vi "HFRR ADV v039.vi"() -> ()   [LabVIEW 2025] (continued)
            n1308 = Not(x=w1623) -> (.not. x?=w1622:bool)
            n1309 = local write "CAMERA ROI MIN TEMP"(w1622) -> ()
            n1310 = call "IMAGE ANALYSIS.vi"("Enum"=POST_ANALYSIS_ENUM."MINIMIZE UI") -> ()  [unwired: 9 in, 2 out]
          }
        }
        n1311 = local write "CAMERA ROI MAX TEMP"(TRUE ("CAMERA ROI MIN TEMP")) -> ()
      }
      frame "Advance" {
        n1312 = local read "LIVE FEED MIN TEMP"() -> (w1629:bool)
        n1313 = local write "LIVE FEED MAX TEMP"(TRUE ("LIVE FEED MAX TEMP")) -> ()
        n1314 = local read "CAMERA ROI MIN TEMP"() -> (w1627:bool)
        n1315 = case shown="True" w1629 {
          selector: w1629 -> [_ w1636]
          frame False {
          }
          frame True {
            n1316 = Not(x=w1636) -> (.not. x?=w1635:bool)
            n1317 = local write "LIVE FEED MIN TEMP"(w1635) -> ()
            n1318 = call "CAMERA LIVE FEED FGV.vi"("Enum - Menu"=CAMERA_LIVE_FEED_ENUM."CAMERA MINIMIZE") -> ()  [unwired: 9 in, 2 out]
          }
        }
        n1319 = local write "CAMERA ROI MAX TEMP"(TRUE ("CAMERA ROI MAX TEMP")) -> ()
        n1320 = case shown="True" w1627 {
          selector: w1627 -> [_ w1633]
          frame False {
          }
          frame True {
            n1321 = Not(x=w1633) -> (.not. x?=w1632:bool)
            n1322 = local write "CAMERA ROI MIN TEMP"(w1632) -> ()
            n1323 = call "IMAGE ANALYSIS.vi"("Enum"=POST_ANALYSIS_ENUM."MINIMIZE UI") -> ()  [unwired: 9 in, 2 out]
          }
        }
      }
      frame "Mooha" {
        n1324 = local read "LIVE FEED MIN TEMP"() -> (w1639:bool)
        n1325 = local write "LIVE FEED MAX TEMP"(TRUE ("LIVE FEED MAX TEMP")) -> ()
        n1326 = local read "CAMERA ROI MIN TEMP"() -> (w1637:bool)
        n1327 = case shown="True" w1639 {
          selector: w1639 -> [_ w1646]
          frame False {
          }
          frame True {
            n1328 = Not(x=w1646) -> (.not. x?=w1645:bool)
            n1329 = local write "LIVE FEED MIN TEMP"(w1645) -> ()
            n1330 = call "CAMERA LIVE FEED FGV.vi"("Enum - Menu"=CAMERA_LIVE_FEED_ENUM."CAMERA MINIMIZE") -> ()  [unwired: 9 in, 2 out]
          }
        }
        n1331 = local write "CAMERA ROI MAX TEMP"(TRUE ("CAMERA ROI MAX TEMP")) -> ()
        n1332 = case shown="True" w1637 {
          selector: w1637 -> [_ w1643]
          frame False {
          }
          frame True {
            n1333 = Not(x=w1643) -> (.not. x?=w1642:bool)
            n1334 = local write "CAMERA ROI MIN TEMP"(w1642) -> ()
            n1335 = call "IMAGE ANALYSIS.vi"("Enum"=POST_ANALYSIS_ENUM."MINIMIZE UI") -> ()  [unwired: 9 in, 2 out]
          }
        }
      }
    }
    n1336 = local read "Auto Start Test"() -> (w1384:bool)
    n1337 = case shown="True" "sign in temp" {
      frame False {
      }
      frame True {
        w1419 = 1 ("y")
        n1338 = local read "USERNAME"() -> (w1425:string)
        n1339 = local read "USER ID"() -> (w1422:string)
        n1340 = call <vilib>:"Trim Whitespace.vi"("string"=w1425) -> ("trimmed string"=w1424:string)  [unwired: 1 in]
        n1341 = call <vilib>:"Trim Whitespace.vi"("string"=w1422) -> ("trimmed string"=w1423:string)  [unwired: 1 in]
        n1342 = String Length(string=w1424) -> (length=w1421:i32)
        n1343 = String Length(string=w1423) -> (length=w1420:i32)
        n1344 = Greater?(x=w1421, y=w1419) -> (0:w1418:bool)
        n1345 = Greater?(x=w1420, y=w1419) -> (0:w1417:bool)
        n1346 = And(x=w1418, y=w1417) -> (x .and. y?=w1416:bool)
        n1347 = case shown="True" w1416 {
          frame False {
            n1348 = property on="Sign In" class="Bool (strict)"("DisabledEnum"=T19."Disabled" ("Disabled")) -> ()  [unwired: 2 in, 2 out]
          }
          frame True {
            n1349 = property on="Sign In" class="Bool (strict)"("DisabledEnum"=T19."Enabled" ("Disabled")) -> ()  [unwired: 2 in, 2 out]
          }
        }
      }
    }
    n1350 = local read "Air Temperature"() -> (w1401:bool)
    n1351 = local read "Coefficient Of Friction"() -> (w1402:bool)
    n1352 = case shown="False" w1384 {
      frame False {
        n1353 = local read "Auto stop temp"() -> (w1413:bool)
        n1354 = case shown="True" w1413 {
          frame False {
          }
          frame True {
            n1355 = local write "Auto Start Temp"(FALSE ("Auto Start Temp")) -> ()
          }
        }
      }
      frame True {
        "Auto stop temp" <- TRUE ("Auto stop temp")
      }
    }
    n1356 = local read "Humidity"() -> (w1400:bool)
    n1357 = case shown="\"HOME\"" w1410 {
      frame "HOME" {
        n1358 = local write "main tab sub"(enum32{"Page 1", "Page 2"}."Page 1" ("main tab sub")) -> ()
      }
      frame Default {
        n1359 = local write "main tab sub"(enum32{"Page 1", "Page 2"}."Page 2" ("main tab sub")) -> ()
      }
    }
    n1360 = case shown="True" w1409 {
      selector: w1409 -> [_ w1761]
      frame False {
      }
      frame True {
        n1361 = Not(x=w1761) -> (.not. x?=w1760:bool)
        n1362 = local write "Sign In"(w1760) -> ()
        n1363 = local write "Main Dashboard Buttons"(T26."Test Setup" ("Main Dashboard Buttons")) -> ()
      }
    }
    n1364 = case shown="\"Numeric Display\", Default" "Num/Graph" {
      frame "Numeric Display", Default {
        n1365 = property on="Single/Multiple" class="RadioBtnsControl (strict)"("Visible"=FALSE) -> ()  [unwired: 2 in, 2 out]
        n1366 = property on="Single - Graph" class="Ring (strict)"("Visible"=FALSE) -> ()  [unwired: 2 in, 2 out]
        n1367 = local write "Main Tab Display"(T4."Dashboard 1" ("Main Tab Display")) -> ()
      }
      frame "Graph Display" {
        n1368 = property on="Single/Multiple" class="RadioBtnsControl (strict)"("Visible"=TRUE) -> ()  [unwired: 2 in, 2 out]
        n1369 = case shown="\"Multiple\"" "Single/Multiple" {
          frame "Single ", Default {
            n1370 = property on="Single - Graph" class="Ring (strict)"("Visible"=TRUE) -> ()  [unwired: 2 in, 2 out]
            n1371 = local write "Main Tab Display"(T4."Dashboard 3" ("Main Tab Display")) -> ()
          }
          frame "Multiple" {
            n1372 = property on="Single - Graph" class="Ring (strict)"("Visible"=FALSE) -> ()  [unwired: 2 in, 2 out]
            n1373 = local write "Main Tab Display"(T4."Dashboard 2" ("Main Tab Display")) -> ()
          }
        }
      }
    }
    n1374 = local read "Stroke"() -> (w1399:bool)
    n1375 = local read "USERNAME"() -> (w1404:string)
    n1376 = case shown="True" w1402 {
      selector: w1402 -> [_ w1686]
      frame False {
      }
      frame True {
        n1377 = Not(x=w1686) -> (.not. x?=w1685:bool)
        n1378 = local write "Coefficient Of Friction"(w1685) -> ()
        n1379 = local write "Tab Control 2"(T6."Coefficient Of Friction" ("Tab Control 2")) -> ()
      }
    }
    n1380 = case shown="True" w1401 {
      selector: w1401 -> [_ w1683]
      frame False {
      }
      frame True {
        n1381 = Not(x=w1683) -> (.not. x?=w1681:bool)
        n1382 = local write "Air Temperature"(w1681) -> ()
        n1383 = local write "Tab Control 2"(T6."Air Temperature" ("Tab Control 2")) -> ()
      }
    }
    n1384 = case shown="True" w1399 {
      selector: w1399 -> [_ w1677]
      frame False {
      }
      frame True {
        n1385 = Not(x=w1677) -> (.not. x?=w1675:bool)
        n1386 = local write "Stroke"(w1675) -> ()
        n1387 = local write "Tab Control 2"(T6."Stroke" ("Tab Control 2")) -> ()
      }
    }
    n1388 = local write "tested by"(w1404) -> ()
    n1389 = case shown="True" w1400 {
      selector: w1400 -> [_ w1680]
      frame False {
      }
      frame True {
        n1390 = Not(x=w1680) -> (.not. x?=w1678:bool)
        n1391 = local write "Humidity"(w1678) -> ()
        n1392 = local write "Tab Control 2"(T6."Humidity" ("Tab Control 2")) -> ()
      }
    }
    n1393 = case shown="\"Calibration\"" "Main Dashboard Buttons" {
      tunnel: [T2."HOME" ("Main Tab") T2."Test Setup" ("Main Tab") T2."Acquire" ("Main Tab") T2."Adv Scar" ("Main Tab") T2."Adv Scar Report" ("Main Tab") T2."Compare Files" ("Main Tab") T2."Calibration" ("Main Tab") T2."About" ("Main Tab") T2."Advance" ("Main Tab")] -> w1383
      frame "Home", Default {
      }
      frame "Test Setup" {
      }
      frame "Dashboard" {
      }
      frame "Imaging" {
      }
      frame "Report" {
      }
      frame "Analysis" {
      }
      frame "Calibration" {
      }
      frame "About" {
      }
      frame "Advance" {
      }
    }
    n1394 = Wait (ms)(milliseconds to wait=u32 100) -> ()  [unwired: 1 out]
    n1395 = local read "Main Tab Display"() -> (w1403:T4)
    n1396 = local write "Main Tab"(w1383) -> ()
    n1397 = case shown="\"Dashboard 3\"" w1403 {
      frame "Dashboard 1", Default {
        n1398 = property on="Reset Graph" class="Bool (strict)"("Visible"=FALSE) -> ()  [unwired: 2 in, 2 out]
      }
      frame "Dashboard 2" {
        n1399 = property on="Reset Graph" class="Bool (strict)"("Visible"=TRUE) -> ()  [unwired: 2 in, 2 out]
      }
      frame "Dashboard 3" {
        n1400 = property on="Reset Graph" class="Bool (strict)"("Visible"=TRUE) -> ()  [unwired: 2 in, 2 out]
      }
    }
    n1401 = local read "SCAR MEASURMENT"() -> (w1391:enum32{"Auto Scar", "Manual Scar"})
    n1402 = local read "Humidity"() -> (w1405:bool)
    n1403 = local read "Cap Live Image"() -> (w1388:bool)
    n1404 = local read "Sample Temperature"() -> (w1398:bool)
    n1405 = local read "Air Temp vs Humidity"() -> (w1396:bool)
    n1406 = local read "Frequency"() -> (w1397:bool)
    n1407 = case shown="False" w1405 {
      frame False {
        n1408 = local write "Humidity On Command"(TRUE ("Humidity On Command")) -> ()
        n1409 = case shown="True" "Humidity Off Command" {
          selector: "Humidity Off Command" -> [_ w1693]
          frame False {
          }
          frame True {
            n1410 = stacked-sequence {
              frame #0 {
                n1411 = local read "WriteHumidity"() -> (w1695:string[])
                n1412 = Insert Into Array(array=w1695, new element="R;1" ("new element/subarray")) -> (w1694:string[])  [unwired: 1 in]
                n1413 = local write "WriteHumidity"(w1694) -> ()
              }
              frame #1 {
                n1414 = Wait (ms)(milliseconds to wait=u32 500) -> ()  [unwired: 1 out]
              }
              frame #2 {
                n1415 = local read "WriteHumidity"() -> (w1699:string[])
                n1416 = local read "EVENT LOG"() -> (w1703:string)
                n1417 = call "Event Log.vi"("Content"="Humidity Control Off" ("string"), "EVENT LOG"=w1703) -> ("EVENT LOG"=w1704:string)  [unwired: 8 in, 1 out]
                n1418 = local write "EVENT LOG"(w1704) -> ()
                n1419 = Insert Into Array(array=w1699, new element="R;1" ("new element/subarray")) -> (w1700:string[])  [unwired: 1 in]
                n1420 = local write "WriteHumidity"(w1700) -> ()
                n1421 = local write "Humidity 2"(TRUE ("Humidity")) -> ()
              }
            }
            n1422 = Not(x=w1693) -> (.not. x?=w1692:bool)
            n1423 = local write "Humidity Off Command"(w1692) -> ()
          }
        }
      }
      frame True {
        n1424 = local write "Humidity Off Command"(TRUE ("Humidity Off Command")) -> ()
        n1425 = case shown="False" "Humidity On Command" {
          selector: "Humidity On Command" -> [_ w1708]
          frame False {
          }
          frame True {
            n1426 = stacked-sequence {
              frame #0 {
                n1427 = local read "Set Rh"() -> (w1714:dbl)
                n1428 = local read "WriteHumidity"() -> (w1710:string[])
                n1429 = Number To Fractional String(number=w1714, precision (6)=i16 2) -> (F-format string=w1715:string)  [unwired: 2 in]
                n1430 = Concatenate Strings("M;" ("new element/subarray"), w1715) -> (w1713:string)
                n1431 = Insert Into Array(array=w1710, new element=w1713) -> (w1709:string[])  [unwired: 1 in]
                n1432 = local write "WriteHumidity"(w1709) -> ()
              }
              frame #1 {
                n1433 = Wait (ms)(milliseconds to wait=u32 500) -> ()  [unwired: 1 out]
              }
              frame #2 {
                n1434 = local read "WriteHumidity"() -> (w1718:string[])
                n1435 = local read "Set Rh"() -> (w1722:dbl)
                n1436 = Number To Fractional String(number=w1722, precision (6)=i16 2) -> (F-format string=w1723:string)  [unwired: 2 in]
                n1437 = Concatenate Strings("M;" ("new element/subarray"), w1723) -> (w1721:string)
                n1438 = Insert Into Array(array=w1718, new element=w1721) -> (w1717:string[])  [unwired: 1 in]
                n1439 = local write "WriteHumidity"(w1717) -> ()
              }
              frame #3 {
                n1440 = Wait (ms)(milliseconds to wait=u32 500) -> ()  [unwired: 1 out]
              }
              frame #4 {
                (unwired) "% RH" ("string")
                (unwired) i16 2 ("precision (6)")
                (unwired) "M;" ("new element/subarray")
                n1441 = local read "Set Rh"() -> (w1732:dbl)
                n1442 = local read "WriteHumidity"() -> (w1725:string[])
                n1443 = Number To Fractional String(number=w1732, precision (6)=i16 2) -> (F-format string=w1729:string)  [unwired: 2 in]
                n1444 = Concatenate Strings("M;" ("new element/subarray"), w1729) -> (w1733:string)
                n1445 = Concatenate Strings("Humidity Set to : " ("string"), w1729, "% RH" ("string")) -> (w1727:string)
                n1446 = Insert Into Array(array=w1725, new element=w1733) -> (w1726:string[])  [unwired: 1 in]
                n1447 = disable-structure shown="Enabled" {
                  frame Enabled {
                    n1448 = local read "EVENT LOG"() -> (w1736:string)
                    n1449 = call "Event Log.vi"("Content"="Humidity Control On", "EVENT LOG"=w1736) -> ("EVENT LOG"=w1737:string)  [unwired: 8 in, 1 out]
                    n1450 = local write "EVENT LOG"(w1737) -> ()
                  }
                  frame Disabled {
                  }
                }
                n1451 = disable-structure shown="Enabled" {
                  disable-tunnel: w1727 -> [_ _]
                  frame Enabled {
                    n1452 = local read "EVENT LOG"() -> (w1739:string)
                    n1453 = call "Event Log.vi"("Content"="Humidity Control On", "EVENT LOG"=w1739) -> ("EVENT LOG"=w1740:string)  [unwired: 8 in, 1 out]
                    n1454 = local write "EVENT LOG"(w1740) -> ()
                  }
                  frame Disabled {
                  }
                }
                n1455 = local write "WriteHumidity"(w1726) -> ()
              }
            }
            n1456 = Not(x=w1708) -> (.not. x?=w1707:bool)
            n1457 = local write "Humidity On Command"(w1707) -> ()
          }
        }
      }
    }
    n1458 = Equal?(x=w1391, y=enum32{"Auto Scar", "Manual Scar"}."Auto Scar" ("SCAR MEASURMENT")) -> (x = y?=w1387:bool)
    n1459 = local read "TEST STANDARD"() -> (w1394:T3)
    n1460 = And(x=w1388, y=w1387) -> (x .and. y?=w1389:bool)
    n1461 = case shown="True" w1389 {
      selector: w1389 -> [_ w1492]
      tunnel: errorcluster {"status"=FALSE, "code"=0, "source"=""} ("error in (no error) 3") -> [_ w1493]
      frame False {
      }
      frame True {
        n1462 = stacked-sequence {
          tunnel: w1493 -> [_ _ _ _ _ _ _ w1541]
          tunnel: w1492 -> [_ _ _ _ _ w1522 _ _]
          frame #0 {
            n1463 = call "CAMERA LIVE FEED FGV.vi"("Enum - Menu"=CAMERA_LIVE_FEED_ENUM."CAMERA MINIMIZE") -> ()  [unwired: 9 in, 2 out]
          }
          frame #1 {
            n1464 = property on="Auto Scar Check  2" class="Clust (strict)"("Visible"=TRUE) -> ()  [unwired: 2 in, 2 out]
          }
          frame #2 {
            n1465 = String To Path(string="C:\\LAB-IQ\\Image Calibrate v01.dcf") -> (path=w1498:path)
            n1466 = Open/Create/Replace File ("Open File")(file path (use dialog)=w1498) -> (refnum out=w1499:refnum<file>)  [unwired: 5 in, 2 out]
            n1467 = for {
              N: 4 -> [_]
              tunnel: w1499 -> [w1505]
              i -> [w1501]
              n1468 = Read from Text File ("Read File")(file (use dialog)=w1505) -> (text=w1506:string)  [unwired: 3 in, 3 out]
              n1469 = String Subset(string=w1506, offset (0)=6, length (rest)=10 ("length (rest)")) -> (substring=w1502:string)
              n1470 = Fract/Exp String To Number(string=w1502) -> (number=w1500:dbl)  [unwired: 3 in, 1 out]
              n1471 = case shown="0" w1501 {
                tunnel: w1500 -> [w1507 w1508 _ w1509 _]
                frame 0 {
                  "5x Gain" <- w1507
                }
                frame 1 {
                  "10x Gain" <- w1508
                }
                frame 2 {
                }
                frame 3 {
                  "100x gain" <- w1509
                }
                frame 4, Default {
                }
              }
            }
          }
          frame #3 {
            n1472 = local read "FILE 3"() -> (w1515:string)
            n1473 = call <vilib>:"Trim Whitespace.vi"("string"="C:\\LAB-IQ\\images\\") -> ("trimmed string"=w1517:string)  [unwired: 1 in]
            n1474 = String To Path(string=w1517) -> (path=w1516:path)
            n1475 = Concatenate Strings(w1515, ".png" ("string")) -> (w1514:string)
            n1476 = Build Path(base path=w1516, name or relative path=w1514) -> (appended path=w1512:path)
            "Image path" <- w1512
            n1477 = Path To String(path=w1512) -> (string=w1511:string)
            n1478 = call "CAMERA LIVE FEED FGV.vi"("Enum - Menu"=CAMERA_LIVE_FEED_ENUM."CAMERA SAVE", "Image Path"=w1511) -> ()  [unwired: 8 in, 2 out]
          }
          frame #4 {
            n1479 = One Button Dialog(message="Image saved successfully") -> ()  [unwired: 1 in, 1 out]
          }
          frame #5 {
            n1480 = local read "TEST STANDARD"() -> (w1521:T3)
            n1481 = local read "Magnification len live scar"() -> (w1533:string)
            n1482 = Not(x=w1522) -> (.not. x?=w1523:bool)
            n1483 = local write "Cap Live Image"(w1523) -> ()
            n1484 = case shown="\"ISO 12156\"" w1521 {
              tunnel: ["ASTM D6079" "ISO 12156"] -> w1520
              frame "ASTM D6079", Default {
              }
              frame "ISO 12156" {
              }
            }
            n1485 = case shown="\"5x\", Default" w1533 {
              tunnel: [w1536 w1537] -> w1532
              frame "5x", Default {
                n1486 = local read "5x Gain"() -> (w1536:dbl)
              }
              frame "10x" {
                # "5x"
                n1487 = local read "10x Gain"() -> (w1537:dbl)
              }
            }
            n1488 = local read "Image path"() -> (w1531:path)
            n1489 = local read "FILE 3"() -> (w1524:string)
            n1490 = call "EDGE DETCTION.vi"("GAIN VALUE"=w1532, "Image Path"=w1531) -> ("error out"=w1530:errorcluster, "return value"=w1529:cluster{string, string, dbl, dbl, dbl})  [unwired: 8 in]
            n1491 = Bundle By Name(cluster=T27 {"File Name"="", "Test Method"="", "Operator"="", "Fuel Description"="", "Date and time"=""} ("Main Ref"), "File Name"=w1524, "Test Method"=w1520) -> (w1525:T27)
            n1492 = call "duf file read.vi"("error in (no error)"=w1530, "Main Ref"=w1525) -> ("error out"=w1528:errorcluster, "Main Ref 2"=w1526:T27)  [unwired: 8 in]
            n1493 = call "EDGE DETECTION REPORT.vi"("error in (no error)"=w1528, "return value 2"=w1529, "Main Ref"=w1526) -> ()  [unwired: 8 in, 1 out]
          }
          frame #6 {
            n1494 = property on="Auto Scar Check  2" class="Clust (strict)"("Visible"=FALSE) -> ()  [unwired: 2 in, 2 out]
          }
          frame #7 {
            n1495 = call "CAMERA LIVE FEED FGV.vi"("Enum - Menu"=CAMERA_LIVE_FEED_ENUM."CAMERA MINIMIZE", "error in (no error)"=w1541) -> ()  [unwired: 8 in, 2 out]
            n1496 = local write "Main Dashboard Buttons"(T1."Home" ("Main Dashboard Buttons")) -> ()
            n1497 = local write "Main Tab"(T2."HOME" ("Main Tab")) -> ()
          }
        }
      }
    }
    n1498 = local read "Heater Button"() -> (w1395:bool)
    n1499 = case shown="True" w1397 {
      selector: w1397 -> [_ w1671]
      frame False {
      }
      frame True {
        n1500 = Not(x=w1671) -> (.not. x?=w1669:bool)
        n1501 = local write "Frequency"(w1669) -> ()
        n1502 = local write "Tab Control 2"(T6."Frequency" ("Tab Control 2")) -> ()
      }
    }
    n1503 = case shown="True" w1396 {
      selector: w1396 -> [_ w1668]
      frame False {
      }
      frame True {
        n1504 = Not(x=w1668) -> (.not. x?=w1666:bool)
        n1505 = local write "Air Temp vs Humidity"(w1666) -> ()
        n1506 = local write "Tab Control 2"(T6."Air Temp vs Rh" ("Tab Control 2")) -> ()
      }
    }
    n1507 = case shown="True" w1398 {
      selector: w1398 -> [_ w1674]
      frame False {
      }
      frame True {
        n1508 = Not(x=w1674) -> (.not. x?=w1672:bool)
        n1509 = local write "Sample Temperature"(w1672) -> ()
        n1510 = local write "Tab Control 2"(T6."Sample Temperature" ("Tab Control 2")) -> ()
      }
    }
    n1511 = case shown="\"Custom\"" w1394 {
      frame "ASTM D6079", Default {
        w1647 = "ASTM D6079 TEST CONDITIONS" ("Standard 2")
        n1512 = local write "Standard 2"(w1647) -> ()
        n1513 = local write "Standard"(w1647) -> ()
      }
      frame "ISO 12156" {
        w1648 = "ISO 12156 TEST CONDITIONS" ("Standard 2")
        n1514 = local write "Standard 2"(w1648) -> ()
        n1515 = local write "Standard"(w1648) -> ()
      }
      frame "CEC F-096-A-06" {
        w1649 = "CEC F-096-A-06 TEST CONDITIONS" ("Standard 2")
        n1516 = local write "Standard 2"(w1649) -> ()
        n1517 = local write "Standard"(w1649) -> ()
      }
      frame "Custom" {
        w1650 = "CUSTOM TEST CONDITIONS" ("Standard 2")
        n1518 = local write "Standard 2"(w1650) -> ()
        n1519 = local write "Standard"(w1650) -> ()
      }
    }
    n1520 = case shown="True" w1395 {
      frame False {
        n1521 = local write "Temperature On Command"(TRUE ("Temperature On Command")) -> ()
        n1522 = case shown="True" "Temperature Off Command" {
          selector: "Temperature Off Command" -> [_ w1654]
          frame False {
          }
          frame True {
            n1523 = Not(x=w1654) -> (.not. x?=w1653:bool)
            n1524 = local read "EVENT LOG"() -> (w1657:string)
            n1525 = local write "Temperature Off Command"(w1653) -> ()
            n1526 = call "Event Log.vi"("Content"="Heater Off", "EVENT LOG"=w1657) -> ("EVENT LOG"=w1656:string)  [unwired: 8 in, 1 out]
            n1527 = local write "EVENT LOG"(w1656) -> ()
          }
        }
      }
      frame True {
        n1528 = local write "Temperature Off Command"(TRUE ("Temperature Off Command")) -> ()
        n1529 = case shown="True" "Temperature On Command" {
          selector: "Temperature On Command" -> [_ w1661]
          frame False {
          }
          frame True {
            n1530 = Not(x=w1661) -> (.not. x?=w1660:bool)
            n1531 = local write "Temperature On Command"(w1660) -> ()
            n1532 = disable-structure shown="Enabled" {
              disable-tunnel: "Heater On" -> [w1663 _]
              frame Enabled {
                n1533 = local read "EVENT LOG"() -> (w1664:string)
                n1534 = call "Event Log.vi"("Content"=w1663, "EVENT LOG"=w1664) -> ("EVENT LOG"=w1665:string)  [unwired: 8 in, 1 out]
                n1535 = local write "EVENT LOG"(w1665) -> ()
              }
              frame Disabled {
              }
            }
          }
        }
      }
    }
    n1536 = local read "Main Tab"() -> (w1386:T2)
    n1537 = case shown="\"About\"" w1386 {
      frame "HOME", Default {
        w1428 = T19."Enabled" ("Disabled")
        n1538 = local read "Service Password enable"() -> (w1430:bool)
        n1539 = property on="Imaging" class="Bool (strict)"("DisabledEnum"=w1428) -> ()  [unwired: 2 in, 2 out]
        n1540 = property on="Dashboard" class="Bool (strict)"("DisabledEnum"=w1428) -> ()  [unwired: 2 in, 2 out]
        n1541 = property on="Test Setup" class="Bool (strict)"("DisabledEnum"=w1428) -> ()  [unwired: 2 in, 2 out]
        n1542 = property on="Analysis" class="Bool (strict)"("DisabledEnum"=w1428) -> ()  [unwired: 2 in, 2 out]
        n1543 = property on="Home" class="Bool (strict)"("DisabledEnum"=w1428) -> ()  [unwired: 2 in, 2 out]
        n1544 = property on="Report" class="Bool (strict)"("DisabledEnum"=w1428) -> ()  [unwired: 2 in, 2 out]
        n1545 = property on="Main Dashboard Buttons" class="RadioBtnsControl (strict)"("DisabledEnum"=w1428) -> ()  [unwired: 2 in, 2 out]
        n1546 = property on="Calibration" class="Bool (strict)"("DisabledEnum"=w1428) -> ()  [unwired: 2 in, 2 out]
        n1547 = case shown="True" w1430 {
          tunnel: [T19."Disabled" ("Disabled") T19."Enabled" ("Disabled")] -> w1429
          frame False {
          }
          frame True {
          }
        }
        n1548 = property on="About" class="Bool (strict)"("DisabledEnum"=w1429) -> ()  [unwired: 2 in, 2 out]
      }
      frame "Test Setup" {
        w1435 = T19."Enabled" ("Disabled")
        n1549 = local read "Service Password enable"() -> (w1434:bool)
        n1550 = property on="Dashboard" class="Bool (strict)"("DisabledEnum"=T19."Disabled" ("Disabled")) -> ()  [unwired: 2 in, 2 out]
        n1551 = property on="Imaging" class="Bool (strict)"("DisabledEnum"=w1435) -> ()  [unwired: 2 in, 2 out]
        n1552 = property on="Analysis" class="Bool (strict)"("DisabledEnum"=w1435) -> ()  [unwired: 2 in, 2 out]
        n1553 = property on="Home" class="Bool (strict)"("DisabledEnum"=w1435) -> ()  [unwired: 2 in, 2 out]
        n1554 = property on="Report" class="Bool (strict)"("DisabledEnum"=w1435) -> ()  [unwired: 2 in, 2 out]
        n1555 = property on="Test Setup" class="Bool (strict)"("DisabledEnum"=w1435) -> ()  [unwired: 2 in, 2 out]
        n1556 = case shown="True" w1434 {
          tunnel: [T19."Disabled" ("Disabled") T19."Enabled" ("Disabled")] -> w1433
          frame False {
          }
          frame True {
          }
        }
        n1557 = property on="About" class="Bool (strict)"("DisabledEnum"=w1433) -> ()  [unwired: 2 in, 2 out]
      }
      frame "Adv Scar" {
        w1442 = T19."Enabled" ("Disabled")
        n1558 = property on="Dashboard" class="Bool (strict)"("DisabledEnum"=T19."Disabled" ("Disabled")) -> ()  [unwired: 2 in, 2 out]
        n1559 = property on="Imaging" class="Bool (strict)"("DisabledEnum"=w1442) -> ()  [unwired: 2 in, 2 out]
        n1560 = property on="Analysis" class="Bool (strict)"("DisabledEnum"=w1442) -> ()  [unwired: 2 in, 2 out]
        n1561 = property on="Home" class="Bool (strict)"("DisabledEnum"=w1442) -> ()  [unwired: 2 in, 2 out]
        n1562 = property on="Report" class="Bool (strict)"("DisabledEnum"=w1442) -> ()  [unwired: 2 in, 2 out]
        n1563 = property on="Test Setup" class="Bool (strict)"("DisabledEnum"=w1442) -> ()  [unwired: 2 in, 2 out]
        n1564 = local read "Service Password enable"() -> (w1440:bool)
        n1565 = case shown="True" w1440 {
          tunnel: [T19."Disabled" ("Disabled") T19."Enabled" ("Disabled")] -> w1439
          frame False {
          }
          frame True {
          }
        }
        n1566 = property on="About" class="Bool (strict)"("DisabledEnum"=w1439) -> ()  [unwired: 2 in, 2 out]
      }
      frame "Calibration" {
        w1445 = T19."Enabled" ("Disabled")
        n1567 = property on="Dashboard" class="Bool (strict)"("DisabledEnum"=T19."Disabled" ("Disabled")) -> ()  [unwired: 2 in, 2 out]
        n1568 = property on="Imaging" class="Bool (strict)"("DisabledEnum"=w1445) -> ()  [unwired: 2 in, 2 out]
        n1569 = property on="Analysis" class="Bool (strict)"("DisabledEnum"=w1445) -> ()  [unwired: 2 in, 2 out]
        n1570 = property on="Home" class="Bool (strict)"("DisabledEnum"=w1445) -> ()  [unwired: 2 in, 2 out]
        n1571 = property on="Report" class="Bool (strict)"("DisabledEnum"=w1445) -> ()  [unwired: 2 in, 2 out]
        n1572 = property on="Test Setup" class="Bool (strict)"("DisabledEnum"=w1445) -> ()  [unwired: 2 in, 2 out]
        n1573 = local read "Service Password enable"() -> (w1447:bool)
        n1574 = property on="Calibration" class="Bool (strict)"("DisabledEnum"=w1445) -> ()  [unwired: 2 in, 2 out]
        n1575 = case shown="True" w1447 {
          tunnel: [T19."Disabled" ("Disabled") T19."Enabled" ("Disabled")] -> w1446
          frame False {
          }
          frame True {
          }
        }
        n1576 = property on="About" class="Bool (strict)"("DisabledEnum"=w1446) -> ()  [unwired: 2 in, 2 out]
      }
      frame "Adv Scar Report" {
        w1453 = T19."Enabled" ("Disabled")
        n1577 = property on="Dashboard" class="Bool (strict)"("DisabledEnum"=T19."Disabled" ("Disabled")) -> ()  [unwired: 2 in, 2 out]
        n1578 = property on="Imaging" class="Bool (strict)"("DisabledEnum"=w1453) -> ()  [unwired: 2 in, 2 out]
        n1579 = property on="Analysis" class="Bool (strict)"("DisabledEnum"=w1453) -> ()  [unwired: 2 in, 2 out]
        n1580 = property on="Home" class="Bool (strict)"("DisabledEnum"=w1453) -> ()  [unwired: 2 in, 2 out]
        n1581 = property on="Report" class="Bool (strict)"("DisabledEnum"=w1453) -> ()  [unwired: 2 in, 2 out]
        n1582 = property on="Test Setup" class="Bool (strict)"("DisabledEnum"=w1453) -> ()  [unwired: 2 in, 2 out]
        n1583 = local read "Service Password enable"() -> (w1452:bool)
        n1584 = case shown="True" w1452 {
          tunnel: [T19."Disabled" ("Disabled") T19."Enabled" ("Disabled")] -> w1451
          frame False {
          }
          frame True {
          }
        }
        n1585 = property on="About" class="Bool (strict)"("DisabledEnum"=w1451) -> ()  [unwired: 2 in, 2 out]
      }
      frame "Compare Files" {
        w1459 = T19."Enabled" ("Disabled")
        n1586 = local read "Service Password enable"() -> (w1458:bool)
        n1587 = property on="Dashboard" class="Bool (strict)"("DisabledEnum"=T19."Disabled" ("Disabled")) -> ()  [unwired: 2 in, 2 out]
        n1588 = property on="Imaging" class="Bool (strict)"("DisabledEnum"=w1459) -> ()  [unwired: 2 in, 2 out]
        n1589 = property on="Analysis" class="Bool (strict)"("DisabledEnum"=w1459) -> ()  [unwired: 2 in, 2 out]
        n1590 = property on="Home" class="Bool (strict)"("DisabledEnum"=w1459) -> ()  [unwired: 2 in, 2 out]
        n1591 = property on="Report" class="Bool (strict)"("DisabledEnum"=w1459) -> ()  [unwired: 2 in, 2 out]
        n1592 = property on="Test Setup" class="Bool (strict)"("DisabledEnum"=w1459) -> ()  [unwired: 2 in, 2 out]
        n1593 = case shown="True" w1458 {
          tunnel: [T19."Disabled" ("Disabled") T19."Enabled" ("Disabled")] -> w1457
          frame False {
          }
          frame True {
          }
        }
        n1594 = property on="About" class="Bool (strict)"("DisabledEnum"=w1457) -> ()  [unwired: 2 in, 2 out]
      }
      frame "Acquire" {
        n1595 = local read "Service Password enable"() -> (w1464:bool)
        n1596 = property on="Test Setup" class="Bool (strict)"("DisabledEnum"=T19."Disabled" ("Disabled")) -> ()  [unwired: 2 in, 2 out]
        n1597 = local read "Auto Start Test"() -> (w1466:bool)
        n1598 = local read "RUN"() -> (w1468:bool)
        n1599 = case shown="True" w1464 {
          tunnel: [T19."Disabled" ("Disabled") T19."Enabled" ("Disabled")] -> w1465
          frame False {
          }
          frame True {
          }
        }
        n1600 = Or(x=w1468, y=w1466) -> (x .or. y?=w1467:bool)
        n1601 = case shown="True" w1467 {
          tunnel: [T19."Enabled" ("Disabled") T19."Disabled" ("Disabled")] -> w1463
          frame False {
          }
          frame True {
          }
        }
        n1602 = property on="About" class="Bool (strict)"("DisabledEnum"=w1465) -> ()  [unwired: 2 in, 2 out]
        n1603 = property on="Imaging" class="Bool (strict)"("DisabledEnum"=w1463) -> ()  [unwired: 2 in, 2 out]
        n1604 = property on="Dashboard" class="Bool (strict)"("DisabledEnum"=w1463) -> ()  [unwired: 2 in, 2 out]
        n1605 = property on="Analysis" class="Bool (strict)"("DisabledEnum"=w1463) -> ()  [unwired: 2 in, 2 out]
        n1606 = property on="Home" class="Bool (strict)"("DisabledEnum"=w1463) -> ()  [unwired: 2 in, 2 out]
        n1607 = property on="Report" class="Bool (strict)"("DisabledEnum"=w1463) -> ()  [unwired: 2 in, 2 out]
        n1608 = property on="Calibration" class="Bool (strict)"("DisabledEnum"=w1463) -> ()  [unwired: 2 in, 2 out]
      }
      frame "About" {
        n1609 = local read "FILE"() -> (w1482:string)
        n1610 = local read "TEST FILE NAM,E SAVED"() -> (w1475:bool)
        n1611 = call <vilib>:"Trim Whitespace.vi"("string"=w1482) -> ("trimmed string"=w1481:string)  [unwired: 1 in]
        n1612 = local read "Auto Start Test"() -> (w1485:bool)
        n1613 = String Length(string=w1481) -> (length=w1480:i32)
        n1614 = Greater?(x=w1480, y=1) -> (0:w1477:bool)
        n1615 = And(x=w1477, y=w1475) -> (x .and. y?=w1476:bool)
        n1616 = local read "RUN"() -> (w1487:bool)
        n1617 = case shown="True" w1476 {
          tunnel: [T19."Disabled" ("Disabled") T19."Enabled" ("Disabled")] -> w1478
          frame False {
          }
          frame True {
          }
        }
        n1618 = Or(x=w1487, y=w1485) -> (x .or. y?=w1486:bool)
        n1619 = property on="About" class="Bool (strict)"("DisabledEnum"=T19."Enabled" ("Disabled")) -> ()  [unwired: 2 in, 2 out]
        n1620 = case shown="False" w1486 {
          tunnel: [T19."Enabled" ("Disabled") T19."Disabled" ("Disabled")] -> w1484
          frame False {
          }
          frame True {
          }
        }
        n1621 = property on="Dashboard" class="Bool (strict)"("DisabledEnum"=w1478) -> ()  [unwired: 2 in, 2 out]
        n1622 = property on="Test Setup" class="Bool (strict)"("DisabledEnum"=T19."Disabled" ("Disabled")) -> ()  [unwired: 2 in, 2 out]
        n1623 = property on="Imaging" class="Bool (strict)"("DisabledEnum"=w1484) -> ()  [unwired: 2 in, 2 out]
        n1624 = property on="Analysis" class="Bool (strict)"("DisabledEnum"=w1484) -> ()  [unwired: 2 in, 2 out]
        n1625 = property on="Home" class="Bool (strict)"("DisabledEnum"=w1484) -> ()  [unwired: 2 in, 2 out]
        n1626 = property on="Report" class="Bool (strict)"("DisabledEnum"=w1484) -> ()  [unwired: 2 in, 2 out]
      }
    }
    n1627 = local read "Quit"() -> (w1412:bool)
    "Single" <- "Single - Graph"
  }
  n1628 = disable-structure shown="Disabled" {
    disable-tunnel: [w1765 _] -> w42
    disable-tunnel: _ -> [w1764 _]
    frame Disabled {
      n1629 = while {
        tunnel: w1764 -> [_]
        tunnel: [w1766] -> w1765
        tunnel: [w1767] -> _
        i -> [w1767]
        stop <- w1766 stop-if-true
        w1783 = u16 10 items=["1.0"=10, "1.5"=15, "2.0"=20] ("stop bits (10: 1 bit)")
        n1630 = Wait (ms)(milliseconds to wait=u32 10) -> ()  [unwired: 1 out]
        n1631 = call-poly "VISA Configure Serial Port"("VISA resource name"=refnum<visa-resource-name> "ASRL1::INSTR" ("COM PORT"), "timeout (10sec)"=u32 10, "baud rate (9600)"=u32 57600, "data bits (8)"=u16 8, "stop bits (10: 1 bit)"=w1783) -> ("VISA resource name out"=w1769:refnum<visa-resource-name>, "error out"=w1778:errorcluster)  [unwired: 9 in]
        n1632 = VISA Read(VISA resource name=w1769, byte count=u32 2 ("byte count (0)")) -> (read buffer=w1777:string)  [unwired: 1 in, 3 out]
        n1633 = String Subset(string=w1777, offset (0)=0, length (rest)=2 ("length (rest)")) -> (substring=w1776:string)
        n1634 = Match Pattern(string=w1776, regular expression="<>") -> (offset past match=w1773:i32)  [unwired: 1 in, 3 out]
        n1635 = Greater Or Equal?(x=w1773, y=0) -> (x >= y?=w1768:bool)
        n1636 = case shown="True" w1768 {
          tunnel: w1769 -> [_ w1787]
          tunnel: w1778 -> [_ w1786]
          frame False {
          }
          frame True {
            n1637 = VISA Read(VISA resource name=w1787, byte count=u32 32 ("byte count (0)"), error in (no error)=w1786) -> (read buffer=w1785:string)  [unwired: 3 out]
            n1638 = String Subset(string=w1785, offset (0)=0, length (rest)=8 ("length (rest)")) -> (substring=w1789:string)
            n1639 = String Subset(string=w1785, offset (0)=8, length (rest)=8 ("length (rest)")) -> (substring=w1790:string)
            n1640 = Decimal String To Number(string=w1790) -> (number=w1797:i32)  [unwired: 2 in, 1 out]
            n1641 = Decimal String To Number(string=w1789) -> (number=w1793:i32)  [unwired: 2 in, 1 out]
            n1642 = Divide(x=w1797, y=10000) -> ()  [unwired: 1 out]
            n1643 = Divide(x=w1793, y=1000000) -> ()  [unwired: 1 out]
          }
        }
        n1644 = local read "Quit"() -> (w1766:bool)
      }
    }
    frame Enabled {
    }
  }
  n1645 = Tick Count (ms)() -> (millisecond timer value=w4:u32)
  n1646 = while {
    shift-right: [w1843] -> _
    shift-left: w6 -> [w1847]
    shift-right: [w1842] -> _
    shift-left: w5 -> [w1846]
    shift-right: [w1841] -> _
    shift-left: w6 -> [w1845]
    shift-right: [w1840] -> _
    shift-left: w5 -> [w1844]
    shift-right: [w1838] -> _
    shift-left: w4 -> [w1839]
    shift-right: [w1835] -> _
    shift-left: w3 -> [w1836]
    shift-right: [w1834] -> _
    shift-left: w3 -> [w1837]
    shift-right: [w1827] -> _
    shift-left: w3 -> [w1833]
    shift-right: [w1826] -> _
    shift-left: w3 -> [w1832]
    shift-right: [w1825] -> _
    shift-left: w3 -> [w1831]
    shift-right: [w1824] -> _
    shift-left: w3 -> [w1830]
    shift-right: [w1823] -> _
    shift-left: w3 -> [w1829]
    shift-right: [w1822] -> _
    shift-left: w3 -> [w1828]
    shift-right: [w1821] -> _
    shift-left: w3 -> [w1815]
    shift-right: [w1820] -> _
    shift-left: w3 -> [w1814]
    shift-right: [w1819] -> _
    shift-left: w3 -> [w1813]
    shift-right: [w1818] -> _
    shift-left: w3 -> [w1812]
    shift-right: [w1817] -> _
    shift-left: w3 -> [w1811]
    shift-right: [w1816] -> _
    shift-left: w3 -> [w1810]
    shift-right: [w1801] -> _
    shift-left: w3 -> [w1804]
    shift-right: [w1800] -> _
    shift-left: w3 -> [w1803]
    shift-right: [w1799] -> _
    shift-left: w3 -> [w1802]
    stop <- w1849 stop-if-true
    n1647 = local read "Read UNO"() -> (w1808:string)
    n1648 = local read "Error  2"() -> (w1848:errorcluster)
    n1649 = String Length(string=w1808) -> (length=w1807:i32)
    n1650 = call <vilib>:"Trim Whitespace.vi"("string"=w1808) -> ("trimmed string"=w1809:string)  [unwired: 1 in]
    n1651 = Greater Or Equal?(x=w1807, y=23) -> (x >= y?=w1805:bool)
    n1652 = case shown="No Error" w1848 {
      tunnel: w1847 -> [w1895 w1991]
      tunnel: w1846 -> [w1894 w1990]
      tunnel: w1845 -> [w1893 w1989]
      tunnel: w1844 -> [w1892 w1988]
      tunnel: [w1891 w1991] -> w1843
      tunnel: [w1890 w1990] -> w1842
      tunnel: [w1889 w1989] -> w1841
      tunnel: [w1888 w1988] -> w1840
      tunnel: w1839 -> [w1887 w1987]
      tunnel: [w1886 w1987] -> w1838
      tunnel: w1836 -> [w1885 w1986]
      tunnel: w1837 -> [w1884 w1985]
      tunnel: [w1883 w1986] -> w1835
      tunnel: [w1882 w1985] -> w1834
      tunnel: w1833 -> [w1881 w1984]
      tunnel: w1832 -> [w1880 w1983]
      tunnel: w1831 -> [w1879 w1982]
      tunnel: w1830 -> [w1878 w1981]
      tunnel: w1829 -> [w1877 w1980]
      tunnel: w1828 -> [w1876 w1979]
      tunnel: [w1875 w1984] -> w1827
      tunnel: [w1874 w1983] -> w1826
      tunnel: [w1873 w1982] -> w1825
      tunnel: [w1872 w1981] -> w1824
      tunnel: [w1871 w1980] -> w1823
      tunnel: [w1870 w1979] -> w1822
      tunnel: w1815 -> [w1869 w1978]
      tunnel: [w1868 w1978] -> w1821
      tunnel: [w1867 w1974] -> w1820
      tunnel: [w1866 w1973] -> w1819
      tunnel: [w1865 w1977] -> w1818
      tunnel: [w1864 w1976] -> w1817
      tunnel: [w1863 w1975] -> w1816
      tunnel: w1814 -> [w1862 w1977]
      tunnel: w1813 -> [w1861 w1976]
      tunnel: w1812 -> [w1860 w1975]
      tunnel: w1811 -> [w1859 w1974]
      tunnel: w1810 -> [w1858 w1973]
      tunnel: w1809 -> [w1857 _]
      tunnel: w1805 -> [w1856 _]
      tunnel: w1804 -> [w1855 w1972]
      tunnel: w1803 -> [w1854 w1971]
      tunnel: w1802 -> [w1853 w1970]
      tunnel: [w1852 w1972] -> w1801
      tunnel: [w1851 w1971] -> w1800
      tunnel: [w1850 w1970] -> w1799
      frame No Error {
        n1653 = case shown="True" w1856 {
          tunnel: w1895 -> [w1911 w1963]
          tunnel: w1894 -> [w1910 w1962]
          tunnel: w1893 -> [w1909 w1961]
          tunnel: w1892 -> [w1908 w1960]
          tunnel: [w1911 w1959] -> w1891
          tunnel: [w1910 w1958] -> w1890
          tunnel: [w1909 w1957] -> w1889
          tunnel: [w1908 w1956] -> w1888
          tunnel: w1887 -> [w1907 w1954]
          tunnel: [w1907 w1953] -> w1886
          tunnel: w1885 -> [w1906 w1952]
          tunnel: w1884 -> [w1905 w1951]
          tunnel: [w1906 w1950] -> w1883
          tunnel: [w1905 w1949] -> w1882
          tunnel: w1881 -> [w1904 w1948]
          tunnel: w1880 -> [w1903 w1947]
          tunnel: w1879 -> [w1902 w1946]
          tunnel: w1878 -> [w1901 w1945]
          tunnel: w1877 -> [w1900 w1944]
          tunnel: w1876 -> [w1899 w1943]
          tunnel: [w1904 w1942] -> w1875
          tunnel: [w1903 w1941] -> w1874
          tunnel: [w1902 w1940] -> w1873
          tunnel: [w1901 w1939] -> w1872
          tunnel: [w1900 w1938] -> w1871
          tunnel: [w1899 w1937] -> w1870
          tunnel: w1869 -> [w1917 w1936]
          tunnel: [w1917 w1935] -> w1868
          tunnel: [w1914 w1934] -> w1867
          tunnel: [w1913 w1933] -> w1866
          tunnel: [w1916 w1932] -> w1865
          tunnel: [w1912 w1931] -> w1864
          tunnel: [w1915 w1930] -> w1863
          tunnel: w1862 -> [w1916 w1929]
          tunnel: w1861 -> [w1915 w1928]
          tunnel: w1860 -> [w1914 w1927]
          tunnel: w1859 -> [w1913 w1926]
          tunnel: w1858 -> [w1912 w1925]
          tunnel: w1857 -> [_ w1924]
          tunnel: w1855 -> [w1898 w1923]
          tunnel: w1854 -> [w1897 w1922]
          tunnel: w1853 -> [w1896 w1921]
          tunnel: [w1898 w1920] -> w1852
          tunnel: [w1897 w1919] -> w1851
          tunnel: [w1896 w1918] -> w1850
          frame False {
          }
          frame True {
            n1654 = Tick Count (ms)() -> (millisecond timer value=w1955:u32)
            n1655 = String To Byte Array(string=w1924) -> (unsigned byte array=w1968:u8[])
            n1656 = Array Size(array=w1968) -> (size(s)=w1967:i32)
            n1657 = formula code="// --- INTERNAL VARIABLE DECLARATIONS ---\nint i = 0;\nint k = 0;\nint start_idx = -1;\nint end_idx = -1;\nint phase = 0;\nint sign0 = 1;\nint sign1 = 1;\nint ch0_val = 0;   \nint ch1_val = 0;   \nfloat ch0_raw = 0.0;\nfloat ch1_raw = 0.0;\nfloat temp0 = 0.0;\nfloat temp1 = 0.0;\nfloat ch0_clean = 0.0;\nfloat ch1_clean = 0.0;\n\nint valid_samples = 0; // FIX: Track if we actually parsed new data this window\nfloat max_allowed_bits = 8388607.0; // FIX: Change this to match your ADC max value\n\n// Temporal intermediate variables for calculation smoothing\nfloat raw_p2p_v = 0.0;\nfloat raw_friction = 0.0;\nfloat raw_cof = 0.0;\n\n// Temporal intermediate variables for Piezo voltage translations\nfloat piezo_min_v = 0.0;\nfloat piezo_max_v = 0.0;\n\n// Initialize output variables to current shift register states right away\nout_LVDT_Min_V = in_LVDT_Min_V;\nout_LVDT_Max_V = in_LVDT_Max_V;\nout_LVDT_P2P_V = in_LVDT_P2P_V;\nout_Piezo_P2P = in_Piezo_P2P;\nout_Friction_N = in_Friction_N;\nout_COF = in_COF;\nwindow_ready = 0;\n\n// --- STEP 1: PARSE EVERY STRING IN THE BYTE ARRAY ---\nif (array_size > 2) {\n    for (i = 0; i < array_size - 1; i++) {\n        if (raw_bytes[i] == 42) { // '*' character detected\n            start_idx = i;\n        }\n        \n        // Match standard delimiter sequence \";&\" or end window character\n        if (raw_bytes[i] == 59 && raw_bytes[i+1] == 38 && start_idx != -1) { \n            end_idx = i;\n            ch0_val = 0;\n            ch1_val = 0;\n            sign0 = 1;\n            sign1 = 1;\n            phase = 0; \n\n            for (k = start_idx + 1; k < end_idx; k++) {\n                if (raw_bytes[k] == 45) { // '-' sign\n                    if (phase == 0) sign0 = -1;\n                    else sign1 = -1;\n                }\n                else if (raw_bytes[k] == 43) { // '+' sign\n                    if (phase == 0) sign0 = 1;\n                    else sign1 = 1;\n                }\n                else if (raw_bytes[k] == 59) { // ';' delimiter\n                    phase = 1; \n                }\n                else if (raw_bytes[k] >= 48 && raw_bytes[k] <= 57) { // Numeric ASCII digits\n                    if (phase == 0) {\n                        ch0_val = (ch0_val * 10) + (raw_bytes[k] - 48);\n                    } else {\n                        ch1_val = (ch1_val * 10) + (raw_bytes[k] - 48);\n                    }\n                }\n            }\n\n            // Implicit type conversion\n            ch0_raw = ch0_val * sign0 * 1.0;\n            ch1_raw = ch1_val * sign1 * 1.0;\n\n            // FIX: Sanity check / Hard-clamping to catch sudden massive ASCII noise spikes\n            if (ch0_raw > max_allowed_bits)  ch0_raw = max_allowed_bits;\n            if (ch0_raw < -max_allowed_bits) ch0_raw = -max_allowed_bits;\n            if (ch1_raw > max_allowed_bits)  ch1_raw = max_allowed_bits;\n            if (ch1_raw < -max_allowed_bits) ch1_raw = -max_allowed_bits;\n\n            // --- STEP 2: 3-SAMPLE MEDIAN FILTER ---\n            m0_2 = m0_1; m0_1 = m0_0; m0_0 = ch0_raw;\n            float s0_0 = m0_0; float s0_1 = m0_1; float s0_2 = m0_2;\n            if (s0_0 > s0_1) { temp0 = s0_0; s0_0 = s0_1; s0_1 = temp0; }\n            if (s0_1 > s0_2) { temp0 = s0_1; s0_1 = s0_2; s0_2 = temp0; }\n            if (s0_0 > s0_1) { temp0 = s0_0; s0_0 = s0_1; s0_1 = temp0; }\n            ch0_clean = s0_1;\n\n            m1_2 = m1_1; m1_1 = m1_0; m1_0 = ch1_raw;\n            float s1_0 = m1_0; float s1_1 = m1_1; float s1_2 = m1_2;\n            if (s1_0 > s1_1) { temp1 = s1_0; s1_0 = s1_1; s1_1 = temp1; }\n            if (s1_1 > s1_2) { temp1 = s1_1; s1_1 = s1_2; s1_2 = temp1; }\n            if (s1_0 > s1_1) { temp1 = s1_0; s1_0 = s1_1; s1_1 = temp1; }\n            ch1_clean = s1_1;\n\n            // --- STEP 3: EXPONENTIAL FILTER (STREAM LEVEL) ---\n            if (ch0_filt == 0.0) ch0_filt = ch0_clean;\n            if (ch1_filt == 0.0) ch1_filt = ch1_clean;\n\n            ch0_filt = ch0_filt + (ch0_clean - ch0_filt) * 0.125;\n            ch1_filt = ch1_filt + (ch1_clean - ch1_filt) * 0.125;\n\n            // --- STEP 4: MIN/MAX WINDOW CONTINUOUS ACCUMULATION ---\n            if (ch0_filt > max_ch0) max_ch0 = ch0_filt;\n            if (ch0_filt < min_ch0) min_ch0 = ch0_filt;\n            if (ch1_filt > max_ch1) max_ch1 = ch1_filt;\n            if (ch1_filt < min_ch1) min_ch1 = ch1_filt;\n\n            valid_samples++; // FIX: Successfully parsed and accumulated a clean point\n            start_idx = -1; \n        }\n    }\n}\n\n// --- STEP 5: WINDOW EVALUATION ENGINE ---\n// FIX: Condition updated to verify that valid samples exist for both channels\nif (((current_time_ms - start_time_ms) >= 50) && (valid_samples > 0) && (min_ch0 < 9000000.0) && (min_ch1 < 9000000.0)) {\n    window_ready = 1;\n\n    // Linear Bit-to-Voltage Transformations (LVDT - Channel 0)\n    out_LVDT_Min_V = (min_ch0 * VREF) / 8388607.0;\n    out_LVDT_Max_V = (max_ch0 * VREF) / 8388607.0;\n    raw_p2p_v = out_LVDT_Max_V - out_LVDT_Min_V;\n\n    // Linear Bit-to-Voltage Transformations (Piezo - Channel 1)\n    piezo_min_v = (min_ch1 * VREF) / 8388607.0;\n    piezo_max_v = (max_ch1 * VREF) / 8388607.0;\n    \n    // Assign Peak-to-Peak Voltage directly to output indicator (Matches Python logic)\n    out_Piezo_P2P = piezo_max_v - piezo_min_v;\n    \n    // Force scaling calculations using Voltage delta * Newtons/Volt Factor\n    raw_friction = out_Piezo_P2P * PIEZO_CAL_FACTOR ;\n    raw_cof = raw_friction / NORMAL_FORCE;\n\n    // --- STEP 6: OUTPUT METRIC SMOOTHING (Low-Pass Filter Alpha = 0.05) ---\n    // Seed initial historical metrics if first loop iteration\n    if (hist_LVDT_P2P == 0.0) hist_LVDT_P2P = raw_p2p_v;\n    if (hist_Friction == 0.0) hist_Friction = raw_friction;\n    if (hist_COF == 0.0)      hist_COF = raw_cof;\n\n    // Apply exponential output dampening\n    hist_LVDT_P2P = hist_LVDT_P2P + (raw_p2p_v - hist_LVDT_P2P) * 0.05;\n    hist_Friction = hist_Friction + (raw_friction - hist_Friction) * 0.05; // Note: Can drop to 0.02 for more aggressive damping\n    hist_COF      = hist_COF + (raw_cof - hist_COF) * 0.05;\n\n    // Direct smoothed parameters out to UI Indicators\n    out_LVDT_P2P_V = hist_LVDT_P2P;\n    out_Friction_N = hist_Friction;\n    out_COF        = hist_COF;\n\n    // Reset tracking targets to extreme boundaries safely\n    min_ch0 = 9999999.0;\n    max_ch0 = -9999999.0;\n    min_ch1 = 9999999.0;\n    max_ch1 = -9999999.0;\n\n    valid_samples = 0; // FIX: Reset counter for next time frame\n    start_time_ms = current_time_ms;\n}"("raw_bytes"=w1968, "array_size"=w1967, "VREF"="VREF", "PIEZO_CAL_FACTOR"="PIEZO_CAL_FACTOR", "NORMAL_FORCE"="NORMAL_FORCE", "min_ch0"=w1963, "max_ch0"=w1962, "min_ch1"=w1961, "max_ch1"=w1960, "current_time_ms"=w1955, "start_time_ms"=w1954, "ch0_filt"=w1952, "ch1_filt"=w1951, "m0_0"=w1948, "m0_1"=w1947, "m0_2"=w1946, "m1_0"=w1945, "m1_1"=w1944, "m1_2"=w1943, "in_LVDT_Min_V"=w1936, "in_LVDT_Max_V"=w1929, "in_LVDT_P2P_V"=w1928, "in_Piezo_P2P"=w1927, "in_Friction_N"=w1926, "in_COF"=w1925, "hist_LVDT_P2P"=w1923, "hist_Friction"=w1922, "hist_COF"=w1921) -> ("window_ready"=→"Valid_data":dbl, "out_LVDT_Min_V"=w1935:dbl, "out_LVDT_Max_V"=w1934:dbl, "out_LVDT_P2P_V"=w1933:dbl, "out_Piezo_P2P"=w1932:dbl, "out_Friction_N"=w1931:dbl, "out_COF"=w1930:dbl, "min_ch0"=w1959:dbl, "max_ch0"=w1958:dbl, "min_ch1"=w1957:dbl, "max_ch1"=w1956:dbl, "start_time_ms"=w1953:u32, "ch0_filt"=w1950:dbl, "ch1_filt"=w1949:dbl, "m0_0"=w1942:dbl, "m0_1"=w1941:dbl, "m0_2"=w1940:dbl, "m1_0"=w1939:dbl, "m1_1"=w1938:dbl, "m1_2"=w1937:dbl, "hist_LVDT_P2P"=w1920:dbl, "hist_Friction"=w1919:dbl, "hist_COF"=w1918:dbl)
            "LVDT MIN" <- w1935
            "LVDT MAX" <- w1934
            "LVDT Peak" <- w1933
            "pizo raw" <- w1932
            "cof" <- w1930
            "Frictioin Force Raw" <- w1931
          }
        }
      }
      frame Error {
      }
    }
    n1658 = local read "Quit"() -> (w1849:bool)
  }
  n1659 = disable-structure shown="Disabled" {
    disable-tunnel: errorcluster {"status"=TRUE, "code"=0, "source"="Init"} ("error IO") -> [w1994 _]
    disable-tunnel: [w1992 _] -> w45
    frame Disabled {
      n1660 = while {
        shift-right: [w2010] -> w1996
        shift-left: _ -> [w2001]
        shift-right: [w2009] -> w1995
        shift-left: w1994 -> [w2003]
        tunnel: [w1998] -> w1992
        tunnel: [w2008] -> _
        i -> [w2008]
        stop <- w1998 stop-if-true
        n1661 = local read "Port 1a"() -> (w2004:bool)
        n1662 = local read "Port 3"() -> (w2005:bool)
        n1663 = local read "Com Port 1"() -> (w2002:refnum<visa-resource-name>)
        n1664 = Or(x=w2005, y=w2004) -> (x .or. y?=w2007:bool)
        n1665 = Unbundle(w2003) -> ("status"=→"Port 3":bool)  [unwired: 2 out]
        n1666 = Not Equal?(x=w2002, y=w2001) -> (x != y?=w1999:bool)
        n1667 = case shown="True" w2007 {
          frame False {
            w2013 = TRUE ("Visible")
            n1668 = property on="Port 1a" class="Bool (strict)"("Visible"=w2013) -> ()  [unwired: 2 in, 2 out]
            n1669 = property on="Port 3" class="Bool (strict)"("Visible"=w2013) -> ()  [unwired: 2 in, 2 out]
          }
          frame True {
            w2014 = TRUE ("Visible")
            n1670 = property on="Port 1a" class="Bool (strict)"("Visible"=w2014) -> ()  [unwired: 2 in, 2 out]
            n1671 = property on="Port 3" class="Bool (strict)"("Visible"=w2014) -> ()  [unwired: 2 in, 2 out]
          }
        }
        n1672 = Wait (ms)(milliseconds to wait=u32 40) -> ()  [unwired: 1 out]
        n1673 = case shown="True" w1999 {
          tunnel: [w2011 errorcluster {"status"=TRUE, "code"=0, "source"="Init"} ("error out")] -> w2000
          tunnel: w2003 -> [w2011 _]
          frame False {
          }
          frame True {
          }
        }
        n1674 = case shown="Error" w2000 {
          selector: w2000 -> [w2021 w2039]
          tunnel: [w2024 w2043] -> w2010
          tunnel: [w2023 w2037] -> w2009
          tunnel: w2001 -> [w2022 w2041]
          frame No Error {
            n1675 = property class="Instr"(reference=w2022, error in=w2021) -> (reference out=w2019:refnum<visa-resource-name>, error out=w2020:errorcluster, "Serial Settings:Number of Bytes at Serial Port"=w2016:u32)
            n1676 = Greater?(x=w2016, y=u32 5) -> (0:w2015:bool)
            n1677 = Not(x=w2015) -> (.not. x?=→"Port 1a":bool)
            n1678 = while {
              tunnel: [w2032] -> w2023
              tunnel: [w2031] -> w2024
              tunnel: w2020 -> [w2030]
              tunnel: w2019 -> [w2029]
              stop <- TRUE stop-if-true
              n1679 = property class="Instr" props=["Serial Settings:Number of Bytes at Serial Port"](reference=w2029, error in=w2030) -> (reference out=w2034:refnum<visa-resource-name>, error out=w2033:errorcluster)  [unwired: 1 out]
              n1680 = VISA Read(VISA resource name=w2034, byte count=u32 50, error in (no error)=w2033) -> (VISA resource name out=w2031:refnum<visa-resource-name>, read buffer=w2026:string, error out=w2032:errorcluster)  [unwired: 1 out]
              n1681 = Wait (ms)(milliseconds to wait=u32 5) -> ()  [unwired: 1 out]
            }
          }
          frame Error {
            w2049 = u16 0 items=["None", "XON/XOFF", "RTS/CTS", "XON/XOFF & RTS/CTS", "DTR/DSR", "XON/XOFF & DTR/DSR"] ("flow control (0:none)  2")
            w2047 = u16 10 items=["1.0"=10, "1.5"=15, "2.0"=20] ("stop bits 2")
            w2045 = u16 0 items=["None", "Odd", "Even", "Mark", "Space"] ("parity 2")
            w2046 = u32 10000  # timeout (10sec)
            n1682 = VISA Close(VISA resource name=w2041, error in (no error)=w2039) -> (error out=w2042:errorcluster)
            n1683 = local write "Port 1a"(FALSE ("Port 1a")) -> ()
            n1684 = local read "Com Port 1"() -> (w2036:refnum<visa-resource-name>)
            n1685 = call <vilib>:"Clear Errors.vi"("error in (no error)"=w2042) -> ("error out"=w2040:errorcluster)  [unwired: 5 in, 1 out]
            n1686 = call-poly "VISA Configure Serial Port"("VISA resource name"=w2036, "timeout (10sec)"=w2046, "baud rate (9600)"=u32 250000 ("baud rate  2"), "data bits (8)"=u16 8 ("data bits  2"), "parity (0:none)"=w2045, "error in (no error)"=w2040, "stop bits (10: 1 bit)"=w2047, "flow control (0:none)"=w2049) -> ("VISA resource name out"=w2050:refnum<visa-resource-name>, "error out"=w2051:errorcluster)  [unwired: 6 in]
            n1687 = flat-sequence {
              tunnel: w2050 -> [w2053]
              tunnel: w2051 -> [w2052]
              tunnel: [w2053] -> w2043
              tunnel: [w2052] -> w2037
              frame #0 {
                n1688 = Wait (ms)(milliseconds to wait=u32 50) -> ()  [unwired: 1 out]
              }
            }
            "Residual Uno" <- ""
          }
        }
        n1689 = local read "Quit"() -> (w1998:bool)
        "Error Uno" <- w2003
      }
      n1690 = VISA Close(VISA resource name=w1996, error in (no error)=w1995) -> (error out=w1993:errorcluster)
      n1691 = call <vilib>:"Clear Errors.vi"("error in (no error)"=w1993) -> ()  [unwired: 5 in, 2 out]
    }
    frame Enabled {
    }
  }
  n1692 = while {
    stop <- w2064 stop-if-true
    # "V0OLTAGE TO STROKE (peice vise calibration)"
    n1693 = local read "LVDT MIN"() -> (w2056:dbl)
    n1694 = local read "LVDT Peak"() -> (w2055:dbl)
    n1695 = Wait (ms)(milliseconds to wait=u32 10) -> ()  [unwired: 1 out]
    n1696 = formula code="// Dynamic Parameterized Linear Interpolation Node\n// Inputs: vpp_val, voltages (Array), distances (Array)\n// Outputs: stroke\n\nint i = 0;\nint segments = 11; // 12 points make 11 interpolation segments\n\n// 1. Lower Boundary Clamp\nif (vpp_val <= voltages[0]) {\n    stroke = distances[0];\n}\n// 2. Upper Boundary Clamp\nelse if (vpp_val >= voltages[segments]) {\n    stroke = distances[segments];\n}\n// 3. Dynamic Segment Search Loop\nelse {\n    stroke = distances[0]; // Fallback baseline\n    for (i = 0; i < segments; i++) {\n        if (vpp_val >= voltages[i] && vpp_val <= voltages[i+1]) {\n            // Standard linear interpolation formula using array lookups\n            stroke = distances[i] + (vpp_val - voltages[i]) * (distances[i+1] - distances[i]) / (voltages[i+1] - voltages[i]);\n            break; // Segment found, safely exit the loop\n        }\n    }\n}"("vpp_val"=w2055, "voltages"="calibration values", "distances"="STROKE") -> ("stroke"=→"LVDT STROKE":dbl)